vi "CaratteristicaDinamica.vi"() -> ()   [LabVIEW 2018]
uses:
  <vilib>/Analysis/baseanly.llb/Mean (DBL).vi
  <vilib>/Analysis/5stat.llb/RMS (DBL).vi
  <vilib>/measure/matone.llb/Extract Single Tone Information 1 Chan.vi
  <vilib>/Analysis/NI_AALPro.lvlib
  <vilib>/measure/NI_MAPro.lvlib
  <vilib>/measure/NI_MABase.lvlib
  <vilib>/Analysis/NI_AALBase.lvlib
panel:
  out "detected frequency":dbl=1000.0053610551311 format="%.2p"
  in  "Tab Control":enum32{"CONFRONTO", "NOISE", "ENOB"}(tab)=enum."ENOB"
  out "Confronto":waveform(dbl)[](graph)=[{"t0"=timestamp(0 s since 1904-01-01), "dt"=9.999999974752427e-07, "Y"=array[1400000 elements]}, {"t0"=timestamp(0 s since 1904-01-01), "dt"=9.999999974752427e-07, "Y"=array[1400000 elements]}]
  out "noise":waveform(dbl)(graph)={"t0"=timestamp(0 s since 1904-01-01), "dt"=9.999999974752427e-07, "Y"=array[1400000 elements]}
  out "ENOB-Freq":cluster{dbl[], dbl[]}(graph)={[10.0, 100.0, 1000.0, 10000.0, 50000.0, 100000.0], [6.52, 6.76, 6.52, 7.71, 5.94, 4.48]}
  out "SNR":dbl=49.64994620708113
  out "ENOB":dbl=6.558584071631862
  in  "length":i32=1400000
  in  "Vertical Coupling (0: A1M)":u16(ring)=2 items=["A1M", "A50", "D1M", "D50", "Ground"]
  in  "Probe Attenuation (1X)":dbl=1.0
  in  "Vertical Range (1 V)":dbl=2.0
  in  "Trigger Level (0.0 V)":dbl
  in  "Timebase (0.0005 s)":dbl=0.1
  in  "Source (1: Channel 1)":u16(ring)=1 items=["Channel 1"=1, "Channel 2"=2, "Channel 3"=3, "Channel 4"=4]
  in  "VISA resource name":refnum<visa-resource-name>="USB0::0xF4EC::0xEE38::SDSMMEBX3R2562::INSTR"
  # "FREQUENZA"
  # "ENOB"
  # "PARAMETRI DELL'ADC"
  # "6.52"
  # "10 Hz"
  # "6.76"
  # "100Hz"
  # "1kHz"
  # "6.52"
  # "10kHz"
  # "7.712"
  # "50kHz"
  # "5.94"
  # "100Hz"
  # "4.48"
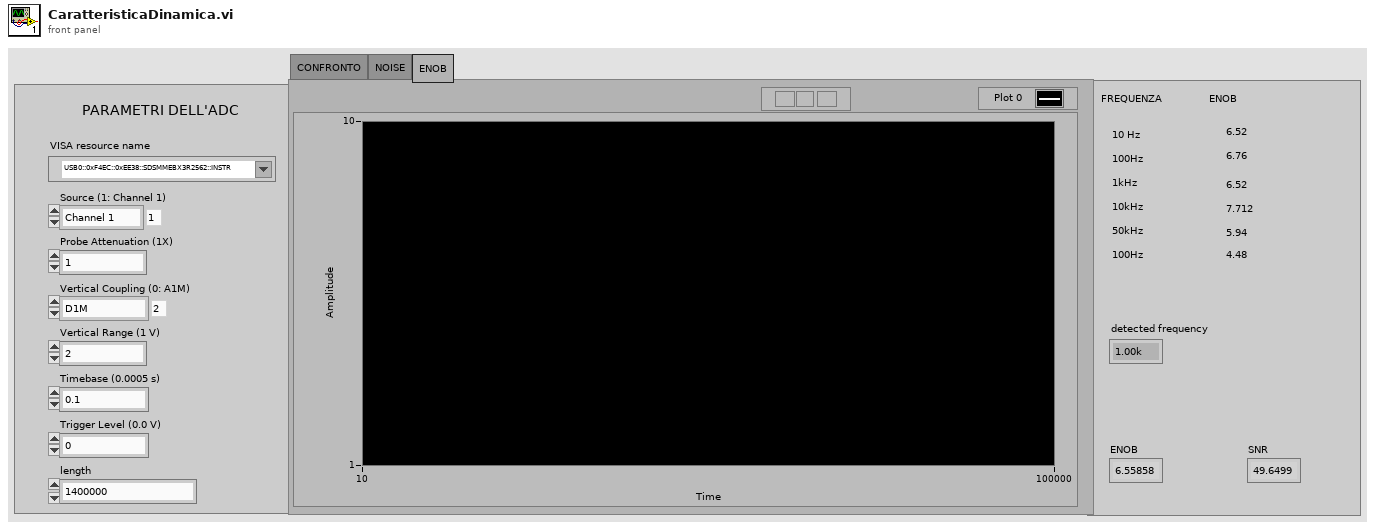
[diagram p1: front panel]
types:
  T1 = enum16{"Sine Wave", "Triangle Wave", "Square Wave", "Sawtooth Wave"}
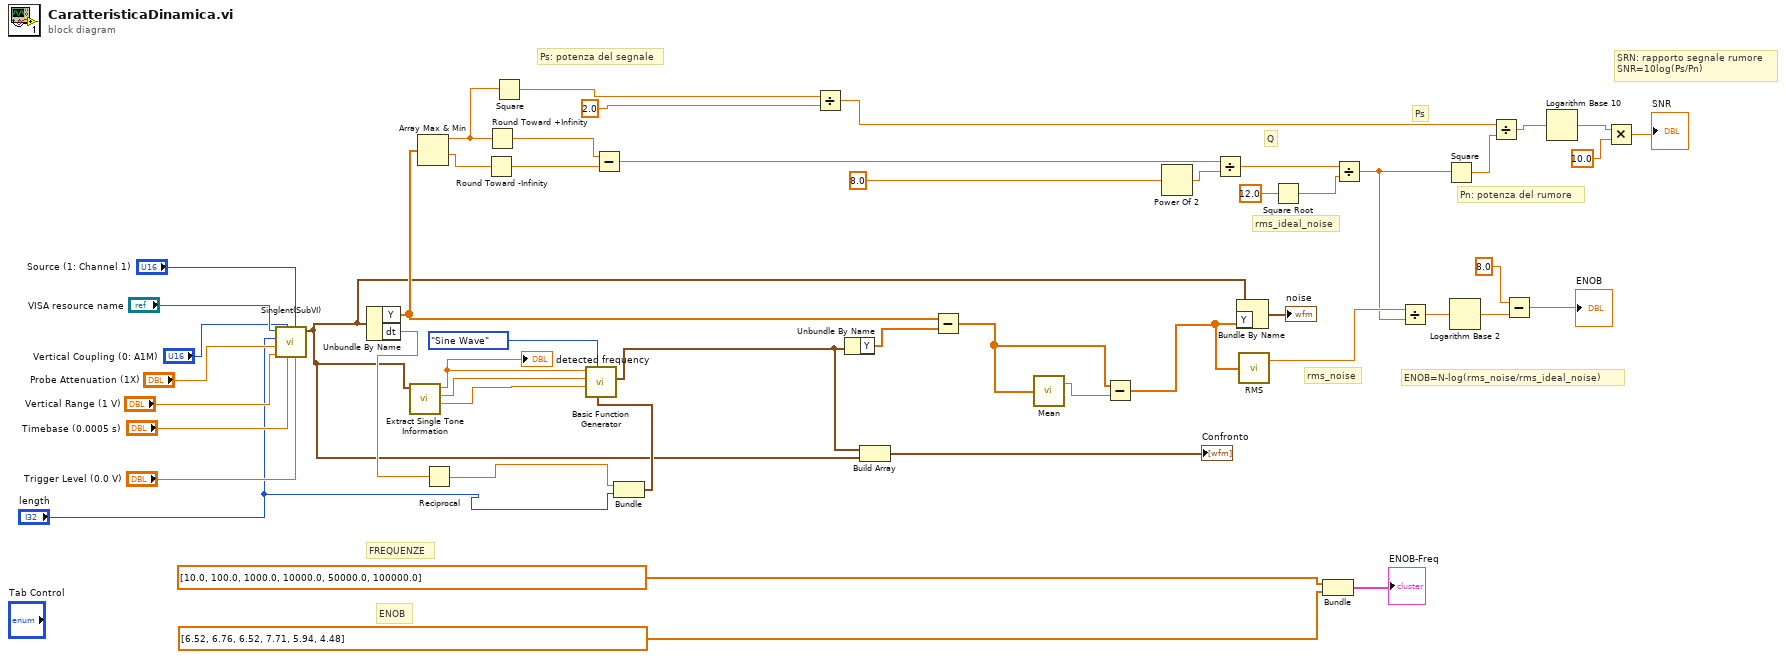
[diagram p0: block diagram]
diagram:
  # "SRN: rapporto segnale rumore\nSNR=10log(Ps/Pn)"
  # "Ps"
  # "Ps: potenza del segnale"
  # "Pn: potenza del rumore"
  # "rms_ideal_noise"
  # "Q"
  # "FREQUENZE"
  # "ENOB"
  # "ENOB=N-log(rms_noise/rms_ideal_noise)"
  # "rms_noise"
  n1 = call "Singlent(SubVI).vi"("Trigger Level (0.0 V)"="Trigger Level (0.0 V)", "Source (1: Channel 1)"="Source (1: Channel 1)", "Timebase (0.0005 s)"="Timebase (0.0005 s)", "Vertical Coupling (0: A1M)"="Vertical Coupling (0: A1M)", "Vertical Range (1 V)"="Vertical Range (1 V)", "Probe Attenuation (1X)"="Probe Attenuation (1X)", "length"="length", "VISA Refnum in"="VISA resource name") -> ("Waveform Graph"=w1:waveform(dbl))  [unwired: 3 in]
  n2 = Unbundle By Name(w1) -> ("Y"=w19:dbl[], "dt"=w8:dbl)
  n3 = call-poly <vilib>:"Extract Single Tone Information.vi"("time signal in"=w1) -> ("detected phase (deg)"=w11:dbl, "detected amplitude"=w12:dbl, "detected frequency"=w13:dbl)  [unwired: 5 in, 3 out]
  "detected frequency" <- w13
  n4 = Array Max & Min(array=w19) -> (max value=w24:dbl, min value=w26:dbl)  [unwired: 2 out]
  n5 = Reciprocal(x=w8) -> (1/x=w6:dbl)
  n6 = Round Toward -Infinity(1:w26) -> (0:w25:dbl)
  n7 = Round Toward +Infinity(x=w24) -> (ceil(x): smallest int >= x=w27:dbl)
  n8 = Square(x=w24) -> (x^2=w23:dbl)
  n9 = Subtract(x=w27, y=w25) -> (x-y=w33:dbl)
  n10 = Bundle(w6, "length"="length") -> (w5:cluster{dbl, "length":i32})  [unwired: 1 in]
  n11 = call <vilib>:"Basic Function Generator.vi"("sampling info"=w5, "signal type"=T1."Sine Wave", "phase"=w11, "amplitude"=w12, "frequency"=w13) -> ("signal out"=w9:waveform(dbl))  [unwired: 4 in, 2 out]
  n12 = Divide(x=w23, y=2.0) -> (x/y=w21:dbl)
  n13 = Unbundle By Name(w9) -> ("Y"=w44:dbl[])
  n14 = Build Array(w9, w1) -> (→"Confronto":waveform(dbl)[])
  n15 = Subtract(x=w19, y=w44) -> (x-y=w3:dbl[])
  n16 = call-poly <vilib>:"Mean.vi"("X"=w3) -> ("mean"=w4:dbl)  [unwired: 1 out]
  n17 = Subtract(x=w3, y=w4) -> (x-y=w2:dbl[])
  n18 = Power Of 2(x=8.0) -> (2^x=w32:dbl)
  n19 = Divide(x=w33, y=w32) -> (x/y=w31:dbl)
  n20 = Bundle By Name(cluster=w1, "Y"=w2) -> (→"noise":waveform(dbl))
  n21 = call-poly <vilib>:"RMS.vi"("X"=w2) -> ("rms value"=w43:dbl)  [unwired: 1 out]
  n22 = Square Root(x=12.0) -> (sqrt(x)=w30:dbl)
  n23 = Bundle(dbl[] [10.0, 100.0, 1000.0, 10000.0, 50000.0, 100000.0], dbl[] [6.52, 6.76, 6.52, 7.71, 5.94, 4.48]) -> (→"ENOB-Freq":cluster{dbl[], dbl[]})  [unwired: 1 in]
  n24 = Divide(x=w31, y=w30) -> (x/y=w18:dbl)
  n25 = Divide(x=w43, y=w18) -> (x/y=w42:dbl)
  n26 = Square(x=w18) -> (x^2=w20:dbl)
  n27 = Logarithm Base 2(1:w42) -> (0:w40:dbl)
  n28 = Divide(x=w21, y=w20) -> (x/y=w15:dbl)
  n29 = Subtract(x=8.0, y=w40) -> (x-y=→"ENOB":dbl)
  n30 = Logarithm Base 10(1:w15) -> (0:w17:dbl)
  n31 = Multiply(x=w17, y=10.0) -> (x*y=→"SNR":dbl)
